vi "View_SUTR_FITS.vi"() -> ()   [LabVIEW 2012]
panel:
  in  "Autosave":bool
  in  "Default Res Directory":path=path "C:/DATA-RESULTS"
  out "error out 2":errorcluster
  in  "Normalize":bool
  in  "FF2":bool
  in  "FF1":bool
  in  "Read 1":bool
  in  "Read 2":bool
  out "Image 2":dbl[][](graph)
  in  "Files 2":i32(listbox)
  in  "Files 1":i32(listbox)
  out "int tome":sgl
  out "Median (ADU/sec)":dbl=6.0 format="%.3f"
  out "file name proc":string="Select file"
  out "Angle 1 ext (deg) 2":dbl=7.5
  out "Angle 1 ext (deg)":dbl=7.5
  out "dV (km/s)":dbl=-1.0193819817582153 format="%.3f"
  out "V (km/s) 2":dbl=7.5
  out "V (km/s) 1":dbl=7.5
  out "Temperature vs refractive index":cluster{dbl[], dbl[]}(graph)
  out "dOrder":dbl=-1.0193819817582153 format="%.3f"
  out "Order 2":dbl=1219.647194648069 format="%.3f"
  out "Order 1":dbl=1219.647194648069 format="%.3f"
  in  "Thickness":dbl=210.0 format="%.3f"
  in  "Wavelength":dbl=1.21 format="%.3f"
  in  "ORDERS/ANGLES":bool
  out "FOCUS 2":dbl[](array[numeric]) format="%.4f"
  out "Image 1":dbl[][](graph)
  in  "HDR PARAM":u16(ring) items=["FOCUS", "Etalons T"]
  out "AXIS 1":cluster{i32[], dbl[]}[](graph)
  out "Array 2":sgl[](array[numeric])
  out "Array":sgl[](array[numeric])
  out "AXIS 3":cluster{i32[], dbl[]}[](graph)
  out "FOCUS":dbl[][](array[numeric]) format="%.4f"
  out "Slice 4":dbl[][](graph)
  in  "Num refpix":u16=5
  in  "Remove refp?":bool
  out "STDEV selected":dbl[][](array[numeric]) format="%.4f"
  in  "Cols  sel":bool[](array[boolean])=[FALSE, TRUE, TRUE, FALSE]
  in  "Rows sel":bool[](array[boolean])=[TRUE, FALSE, FALSE, TRUE]
  out "Slice 3":dbl[][](graph)
  out "Slice 2":dbl[][](graph)
  in  "Init params colS":T1(array[cluster])=[{"initial amplitude"=33.77719364785919, "initial center"=49.70463978212081, "initial std devi"=0.19273176170627804, "offset"=90.64950374672406}, {"initial amplitude"=2584.714260893242, "initial center"=65.44858138705881, "initial std devi"=3.733463983192803, "offset"=284.499091020463}, {"initial amplitude"=780.252289907369, "initial center"=76.39143911404652, "initial std devi"=10.23938098152215, "offset"=81.40579465327467}, {"initial amplitude"=500.0, "initial center"=50.0, "initial std devi"=5.0, "offset"=0.0}]
  in  "Init params ROW":T1(array[cluster])=[{"initial amplitude"=1873.6125304433974, "initial center"=69.54989529124263, "initial std devi"=4.504262475173647, "offset"=252.28578992831524}, {"initial amplitude"=19.137742970969033, "initial center"=37.10397468007118, "initial std devi"=78.15537278387357, "offset"=38.82421297074018}, {"initial amplitude"=19.04875576622036, "initial center"=99.0, "initial std devi"=197.98265411656024, "offset"=62.014220893292794}, {"initial amplitude"=1000.0, "initial center"=50.0, "initial std devi"=5.0, "offset"=0.0}]
  in  "files":string[](array[string])
  in  "Read":bool
  out "Amplitude 2":dbl[][](array[numeric]) format="%.4f"
  out "STDEV 2":dbl[][](array[numeric]) format="%.4f"
  out "center 2":dbl[][](array[numeric]) format="%.4f"
  in  "initial guess COL":T2={"initial amplitude"=nan, "initial center"=nan, "initial std devi"=nan, "offset"=nan}
  out "center":dbl[][](array[numeric]) format="%.4f"
  out "STDEV":dbl[][](array[numeric]) format="%.4f"
  out "Amplitude":dbl[][](array[numeric]) format="%.4f"
  in  "error in (no error)":errorcluster
  in  "Process":bool
  in  "STOP":bool
  in  "Strip length":i32=600
  in  "Fit Gauss?":bool
  out "proc file #":i32
  in  "Select flatfield":u16(ring) items=["Std", "Read from disk", "Average  files"]
  in  "Norm?":bool
  out "Slice 7":dbl[][](graph)
  in  "FF array":dbl[][](array[numeric])=array1024x1024[1048576 elements] format="%.4f"
  out "Slice 6":dbl[][](graph)
  in  "Select file":string="Select file"
  out "Numeric":i32=3
  out "STDEV":dbl[][](graph)=[[3.80922583304428, 3.817188088612178, 3.977756374635943, 3.709975839173165, 4.204670281550964, 4.066080878455446, 4.561354633571724, 4.5262390212577985, 4.558772835455342, 4.581136884063742, 4.521486316852289, 4.971843226595924, 4.90608258535995, 5.27696401550079, 5.111911508066236, 5.170141203091181, 4.890928111688745, 4.907247135437398, 4.848191242418806, 4.83809156293769], [9.711095280614401, 9.971289019821658, 9.788245843410733, 9.923357541329326, 9.745666322543594, 9.786236649177065, 9.511348120785584, 9.373091410919924, 9.304927522805341, 9.10012745113379, 9.146622952912985, 8.993768484218087, 8.956214514109512, 8.674866890194615, 8.719154141237079, 8.611851720736974, 7.701630409119083, 7.651212652849094, 7.609036134707259, 7.603366762011219], [4.893862283261521, 3.912348921910702, 4.287711111176547, 3.968009269163568, 4.42781957244485, 4.444836685027503, 4.741397672118246, 4.721056037339747, 4.626346526841245, 4.919177778951065, 5.100781252748569, 5.5392420746888495, 5.539933224601394, 5.6020059507282385, 5.808813620501355, 6.182585147680958, 5.756524829207016, 5.473299468339225, 5.511785993835031, 5.18370376288494], [9.258933828121483, 9.191747417698833, 9.041217540948582, 9.413425961872695, 8.829487668253286, 9.160443411114333, 9.114654291796361, 8.72041762857734, 8.959900586090964, 8.636980944545334, 9.046089389007006, 8.887693711855636, 8.875586055417067, 8.921953916385833, 8.9718505032208, 9.04963948163129, 9.904011705941352, 9.675772758013501, 9.638785423011441, 9.552602582469593]]
  in  "parameter bounds":T3={"amp min"=0.0, "amp max"=20000.0, "center min"=0.0, "center max"=200.0, "deviation min"=-inf, "deviation max"=100.0, "offset min"=0.0, "offset max"=20000.0}
  out "STDV":dbl=9.552602582469593
  out "Position":dbl=49.896376621079575
  out "Amplitude":dbl=1955.4840499678983
  in  "Selection length":i32=200
  out "Slice 4":dbl[](graph)
  in  "initial guess ROW":T2={"initial amplitude"=nan, "initial center"=nan, "initial std devi"=nan, "offset"=nan}
  out "STDV":dbl[][](array[numeric])=[[3.80922583304428, 9.711095280614401, 4.893862283261521, 9.258933828121483], [3.817188088612178, 9.971289019821658, 3.912348921910702, 9.191747417698833], [3.977756374635943, 9.788245843410733, 4.287711111176547, 9.041217540948582], [3.709975839173165, 9.923357541329326, 3.968009269163568, 9.413425961872695], [4.204670281550964, 9.745666322543594, 4.42781957244485, 8.829487668253286], [4.066080878455446, 9.786236649177065, 4.444836685027503, 9.160443411114333], [4.561354633571724, 9.511348120785584, 4.741397672118246, 9.114654291796361], [4.5262390212577985, 9.373091410919924, 4.721056037339747, 8.72041762857734], [4.558772835455342, 9.304927522805341, 4.626346526841245, 8.959900586090964], [4.581136884063742, 9.10012745113379, 4.919177778951065, 8.636980944545334], [4.521486316852289, 9.146622952912985, 5.100781252748569, 9.046089389007006], [4.971843226595924, 8.993768484218087, 5.5392420746888495, 8.887693711855636], [4.90608258535995, 8.956214514109512, 5.539933224601394, 8.875586055417067], [5.27696401550079, 8.674866890194615, 5.6020059507282385, 8.921953916385833], [5.111911508066236, 8.719154141237079, 5.808813620501355, 8.9718505032208], [5.170141203091181, 8.611851720736974, 6.182585147680958, 9.04963948163129], [4.890928111688745, 7.701630409119083, 5.756524829207016, 9.904011705941352], [4.907247135437398, 7.651212652849094, 5.473299468339225, 9.675772758013501], [4.848191242418806, 7.609036134707259, 5.511785993835031, 9.638785423011441], [4.83809156293769, 7.603366762011219, 5.18370376288494, 9.552602582469593]]
  out "Peak position":dbl[][](array[numeric])=[[47.66372822279346, 45.737706176461124, 32.064423476273895, 41.26378980520465], [48.037887071447074, 44.121616415233404, 29.0359957584797, 42.88856881625823], [47.46412751971739, 43.40189101127855, 28.315113746919998, 42.853423144990614], [47.23633903151997, 43.98331127448147, 28.17624968549179, 43.20820023705084], [47.11670684274625, 43.43988511102371, 27.74805501482961, 43.138657897597355], [46.93922903400806, 43.9466885921773, 27.747501552953953, 43.29781271217172], [46.983170601290446, 43.4674057822943, 27.349010989971706, 43.4928736930594], [46.87826650279293, 43.73656484581372, 27.231418867922137, 43.59027544271928], [46.794602213066604, 43.80697609235037, 27.219441141475325, 43.86228314076525], [46.547609840673196, 43.49560932641496, 26.737210482499357, 43.83683218582205], [46.50275300580495, 43.93616768488781, 26.586165471065954, 44.24335733899606], [46.3894955614418, 43.74599122414512, 26.43758155462442, 44.18898136177602], [46.216839101721845, 44.127049565224574, 25.990860317183685, 44.52332837815359], [46.17676540353349, 43.92341806193053, 25.796393903324972, 44.59364842655686], [45.94651003970945, 44.243386449383074, 25.67343920426777, 44.94522728573687], [46.038982620545305, 43.96184867410636, 25.099486713825282, 45.28759471092761], [42.07400933436385, 46.63026758012912, 20.913656675675835, 49.256809286246366], [41.8831791471293, 46.71508407353966, 20.458660051313952, 49.58491224283602], [41.70930139549427, 46.95675849721172, 20.21435561030008, 49.95477829486535], [41.571263488082245, 46.859185888986325, 20.01183300897636, 49.896376621079575]]
  out "Amplitude":dbl[][](array[numeric])=[[2105.8622124215794, 1639.2467702622673, 2142.5270817793817, 1911.2610434851829], [2120.0504394951727, 1630.518269247327, 2157.8793469310863, 1968.0887445364817], [2074.081974979694, 1636.7175569641458, 2051.291440379497, 2013.3151234716927], [2141.4467291327323, 1637.469594377443, 2097.2888406416005, 1963.261978839169], [2066.222742080296, 1675.75453156014, 1978.306748333681, 2039.902099411284], [2067.624264099335, 1649.5982827860123, 1974.9594809186055, 2007.8700226013175], [1930.3219711177662, 1671.664946884232, 1963.7304764864682, 1990.0291865018387], [1934.7065510066398, 1695.403255048172, 1857.3519938646368, 2087.6349072163557], [2010.3064992166367, 1739.9324821026587, 1938.6975619656757, 2061.5356631230625], [1973.3790444228753, 1724.343555695147, 1890.962522743408, 2092.6867904284627], [1919.5387889965712, 1717.728353100013, 1795.3689110727476, 2025.044521524015], [1903.7560193442341, 1721.9496201330182, 1766.6216531350074, 2048.568854184652], [1930.4201947084764, 1755.9174293651708, 1799.1996079210312, 2065.114852823516], [1839.8756755419372, 1800.8508402487678, 1770.4507853937826, 2097.8006996715453], [1809.800026316876, 1800.6809656752282, 1725.998803512788, 2064.175733682101], [1803.9896118206118, 1802.8721092945568, 1680.5647072776162, 2085.0002611575646], [1908.2524607314188, 1994.827370627359, 1648.1186318102089, 1950.312562150539], [1902.2584452330298, 1968.3910778062084, 1640.241397396131, 1941.6845145841237], [1893.25547881938, 1983.5729978506592, 1613.927881985334, 1942.0488428956264], [1910.0015420712516, 1975.1048979055772, 1628.0987604984884, 1955.4840499678983]]
  out "Number of files":i32=20
  in  "Flatfield?":bool
  out "Sub Array":i32[][](array[numeric])
  out "Header":string="SIMPLE  =                    T / Files does conform to FITS standard            BITPIX  =                  -32 / Number of bits per data pixel                  NAXIS   =                    2 / Number of data axes                            NAXIS1  =                 1024 / Length of data axis 1                          NAXIS2  =                 1024 / Length of data axis 2                          EXTEND  =                      / FITS dataset may contain extensions            FOWLERNU=                    1 / Number of Fowler pairs                         OBJECT  =                      / Object Name                                    TELESCOP=                      / Telescope Name                                 INSTRUME=               'ZODI' / Instrument Name                                OBSERVER=                      / Observer Name                                  EQUINOX =                      / Coordinate Epoch                               NAME    ='111030412.5622.fits' / Filename                                       DATE    =         '03/04/2011' / Date                                           TIME    =           '12:56:22' / Time                                           JULIAN  =        2455625.24748 / Julian Date                                    INTTIME =             1.000000 / Integration Time                               FILTER  =                      / Filter                                         BSCALE  =                  1.0 / B Scale                                        BZERO   =                  0.0 / B Zero                                         CTYPE1  =             'PIXELS' / Axis type for dim 1 (e.g. RA)                  CTYPE2  =             'PIXELS' / Axis type for dim 2 (e.g. DEC)                 CRVAL1  =              0.00000 / Sky coord of 1st axis RA  (deg)                CRVAL2  =              0.00000 / Sky coord of 2nd axis DEC (deg)                CRPIX1  =                      / RA  ref point pixel location                   CRPIX2  =                      / DEC ref point pixel location                   TEMPA   =                 0.00 / Channel A                                      TEMPB   =                 0.00 / Channel B                                      TEMPC1  =                 0.00 / Etalon 1-250                                   TEMPC2  =                 0.00 / Etalon 2-210                                   TEMPC3  =                 0.00 / Filter Box                                     TEMPC4  =                 0.00 / Cold Plate                                     TEMPD1  =                 0.00 / Detector                                       TEMPD2  =                 0.00 / none                                           TEMPD3  =                 0.00 / none                                           TEMPD4  =                 0.00 / none                                           BIAS1   =                4.010 / BIAS 1                                         BIAS2   =                3.922 / BIAS 2                                         BIAS3   =                4.012 / BIAS 3                                         BIAS4   =                3.991 / BIAS 4                                         BIAS5   =                4.000 / BIAS 5                                         BIAS6   =                4.000 / BIAS 6                                         BIAS7   =                4.000 / BIAS 7                                         BIAS8   =                4.000 / BIAS 8                                         FOCUS1  =               -1.391 / Focus X Position                               FOCUS2  =                0.173 / Focus Y Position                               FOCUS3  =                0.020 / Focus Z Position                               FLTINDX =                    0 / Filter Index                                   FLTSTEP =                    0 / Filter Steps                                   FNAME   =                      / Filter Name                                    PRESSURE=          0.000000E+0 / Pressure                                       HEAT1   =                0.000 / Heater Etalon 1                                HEAT2   =                0.000 / Heater Etalon 2                                HEATD   =                0.000 / Heater Detector                                COMMENT =                                                                       END                                                                             "
  in  "Strip width":i32=20
  out "Slice 1":dbl[][](graph)
  out "Slice 2":dbl[](graph)=[-306.0, 4.0, -8.0, 11.0, -8.0, 226.0, 150.0, 188.0, 141.0, 154.0, 207.0, 167.0, 233.0, 226.0, 240.0, 292.0, 266.0, 288.0, 310.0, 280.0, 282.0, 336.0, 316.0, 206.0, 352.0, 136.0, 228.0, 300.0, 225.0, 284.0, 171.0, 136.0, 119.0, 150.0, 117.0, 114.0, 146.0, 142.0, 132.0, 102.0, 104.0, 113.0, 98.0, 110.0, 116.0, 70.0, 60.0, 66.0, 150.0, 132.0, 88.0, 96.0, 96.0, 138.0, 96.0, 185.0, 99.0, 98.0, 133.0, 110.0, 77.0, 74.0, 58.0, 72.0, 151.0, 106.0, 73.0, 116.0, 148.0, 150.0, 84.0, 98.0, 131.0, 122.0, 49.0, 128.0, 80.0, 80.0, 129.0, 165.0, 117.0, 107.0, 153.0, 118.0, 100.0, 97.0, 132.0, 181.0, 107.0, 105.0, 132.0, 138.0, 100.0, 69.0, 126.0, 118.0, 56.0, 94.0, 91.0, 119.0, 70.0, 86.0, 68.0, 108.0, 117.0, 176.0, 72.0, 102.0, 120.0, 138.0, 114.0, 130.0, 98.0, 121.0, 134.0, 103.0, 127.0, 109.0, 119.0, 210.0, 148.0, 134.0, 169.0, 122.0, 116.0, 126.0, 152.0, 92.0, 96.0, 218.0, 168.0, 228.0, 199.0, 197.0, 81.0, 168.0, 186.0, 169.0, 219.0, 184.0, 231.0, 200.0, 298.0, 296.0, 384.0, 262.0, 288.0, 514.0, 462.0, 442.0, 444.0, 342.0, 446.0, 592.0, 631.0, 696.0, 537.0, 796.0, 1097.0, 1056.0, 1286.0, 1415.0, 2354.0, 1398.0, 1502.0, 1508.0, 2106.0, 1889.0, 2272.0, 1350.0, 1890.0, 2253.0, 2489.0, 2663.0, 1860.0, 1565.0, 1630.0, 1408.0, 1197.0, 1240.0, 1414.0, 1125.0, 998.0, 932.0, 1024.0, 727.0, 776.0, 843.0, 627.0, 540.0, 442.0, 447.0, 413.0, 403.0, 308.0, 246.0, 302.0, 325.0, 389.0, 327.0, 244.0, 342.0, 235.0, 270.0, 350.0, 312.0, 232.0, 332.0, 240.0, 306.0, 210.0, 186.0, 236.0, 179.0, 216.0, 180.0, 240.0, 132.0, 249.0, 185.0, 194.0, 219.0, 109.0, 268.0, 301.0, 117.0, 167.0, 183.0, 64.0, 106.0, 174.0, 146.0, 161.0, 99.0, 114.0, 147.0, 93.0, 171.0, 120.0, 100.0, 165.0, 144.0, 216.0, 145.0, 75.0, 85.0, 108.0, 110.0, 158.0, 75.0, 128.0, 102.0, 150.0, 138.0, 101.0, 135.0, 104.0, 240.0, 157.0, 112.0, 115.0, 80.0, 76.0, 81.0, 127.0, 114.0, 82.0, 98.0, 110.0, 140.0, 116.0, 119.0, 145.0, 89.0, 176.0, 107.0, 214.0, 141.0, 61.0, 120.0, 118.0, 140.0, 112.0, 103.0, 30.0, 125.0, 151.0, 150.0, 162.0, 126.0, 92.0, 115.0, 73.0, 158.0, 150.0, 111.0, 124.0, 146.0, 81.0, 284.0, 154.0, 169.0, 155.0, 138.0, 124.0, 153.0, 96.0, 178.0, 170.0, 130.0, 139.0, 122.0, 103.0, -37.0, 122.0, 155.0, 106.0, 65.0, 79.0, 102.0, 117.0, 92.0, 64.0, 95.0, 96.0, 11.0, 116.0, 95.0, 119.0, 108.0, 63.0, 197.0, 118.0, 62.0, 50.0, 82.0, 77.0, 178.0, 110.0, 71.0, 62.0, 100.0, 75.0, 125.0, 70.0, 100.0, 148.0, 125.0, 97.0, 119.0, 140.0, 82.0, 144.0, 126.0, 74.0, 64.0, 62.0, 116.0, 90.0, 93.0, 110.0, 60.0, 84.0, 141.0, 43.0, 42.0, 90.0, 140.0, 98.0, 58.0, 119.0, 103.0, 136.0, 138.0, 70.0, 103.0, 115.0, 82.0, 97.0, 98.0, 100.0, 68.0, 105.0, 99.0, 84.0, 77.0, 88.0, 94.0, 192.0, 79.0, 131.0, 112.0, 88.0, 131.0, 62.0, 96.0, 148.0, 81.0, 108.0, 53.0, 75.0, 124.0, 111.0, 116.0, 137.0, 67.0, 113.0, 96.0, 60.0, 46.0, 119.0, 98.0, 130.0, 137.0, 178.0, 82.0, 43.0, 116.0, 143.0, 116.0, 107.0, 146.0, 121.0, 100.0, 101.0, 150.0, 155.0, 106.0, 75.0, 65.0, 92.0, 84.0, 68.0, 102.0, 98.0, 64.0, 123.0, 82.0, 109.0, 106.0, 101.0, 68.0, 95.0, 88.0, 97.0, 92.0, 79.0, 98.0, 57.0, 117.0, 89.0, 146.0, 41.0, 110.0, 85.0, 110.0, 134.0, 152.0, 60.0, 90.0, 183.0, 102.0, 110.0, 98.0, 144.0, 178.0, 144.0, 67.0, 119.0, 72.0, -25.0, 128.0, 78.0, 127.0, 105.0, 84.0, 91.0, 12.0, 93.0, 128.0, 157.0, 81.0, 48.0, 119.0, 115.0, 98.0, 123.0, 109.0, 94.0, 83.0, 74.0, 96.0, 148.0, 104.0, 123.0, 82.0, 46.0, 87.0, 74.0, 91.0, 54.0, 116.0, 147.0, 72.0, 157.0, 66.0, 110.0, 118.0, 60.0, 82.0, 126.0, 124.0, 124.0, 75.0, 138.0, 102.0, 92.0, 122.0, 58.0, 76.0, 63.0, 95.0, 74.0, 114.0, 88.0, 114.0, 56.0, 106.0, 89.0, 104.0, 68.0, 60.0, 121.0, 129.0, 118.0, 74.0, 188.0, 203.0, 162.0, 180.0, 81.0, 131.0, 77.0, 38.0, 66.0, 113.0, 139.0, 101.0, 113.0, 83.0, 70.0, 89.0, 103.0, 87.0, 86.0, 95.0, 78.0, 104.0, 148.0, 98.0, 62.0, 108.0, 52.0, 121.0, 112.0, 126.0, 68.0, 110.0, 77.0, 186.0, 117.0, 111.0, 103.0, 109.0, 157.0, 120.0, 116.0, 49.0, 12.0, 84.0, 144.0, 64.0, 72.0, 90.0, 86.0, 122.0, 41.0, 102.0, 96.0, 145.0, 112.0, 56.0, 58.0, 103.0, 114.0, 85.0, 58.0, 72.0, 67.0, 155.0, 62.0, 80.0, 137.0, 70.0, 98.0, 76.0, 98.0, 113.0, 125.0, 112.0, 107.0, 140.0, 84.0, 95.0, 80.0, 95.0, 96.0, 131.0, 88.0, 108.0, 48.0, 64.0, 115.0, 69.0, 76.0, 154.0, 138.0, 79.0, 129.0, 122.0, 139.0, 89.0, 86.0, 143.0, 123.0, 104.0, 53.0, 82.0, 152.0, 102.0, 57.0, 119.0, 120.0, 74.0, 132.0, 63.0, 86.0, 125.0, 95.0, 110.0, 136.0, 81.0, 91.0, 97.0, 82.0, 63.0, 154.0, 123.0, 110.0, 79.0, 54.0, 104.0, 180.0, 102.0, 50.0, 144.0, 111.0, 42.0, 84.0, 99.0, 126.0, 73.0, 101.0, 116.0, 85.0, 107.0, 89.0, 37.0, 98.0, 112.0, 79.0, 106.0, 103.0, 179.0, 102.0, 78.0, 125.0, 104.0, 97.0, 84.0, 88.0, 136.0, 32.0, 79.0, 102.0, 84.0, 34.0, 108.0, 76.0, 38.0, 134.0, 69.0, 81.0, 103.0, 85.0, 129.0, 143.0, 71.0, 98.0, 94.0, 44.0, 81.0, 175.0, 35.0, 118.0, 84.0, 179.0, 89.0, 37.0, 90.0, 87.0, 84.0, 88.0, 46.0, 36.0, 92.0, 76.0, 68.0, 54.0, -39.0, 60.0, 45.0, 68.0, 88.0, 128.0, 160.0, 121.0, 60.0, 124.0, 49.0, 122.0, 109.0, 174.0, 103.0, 95.0, 105.0, 134.0, 77.0, 77.0, 78.0, 141.0, 36.0, 74.0, 121.0, 88.0, 74.0, 95.0, 110.0, 105.0, 174.0, 68.0, 136.0, 128.0, 66.0, 70.0, 40.0, 72.0, 92.0, 95.0, 97.0, 49.0, 153.0, 109.0, 70.0, 62.0, 60.0, 158.0, 79.0, 92.0, 161.0, 66.0, 67.0, 78.0, 96.0, 109.0, 51.0, 173.0, 108.0, 147.0, 183.0, 74.0, 94.0, 120.0, 80.0, 134.0, 89.0, 56.0, -16.0, 94.0, 90.0, 26.0, 124.0, 88.0, 88.0, 82.0, 56.0, 67.0, 93.0, 104.0, 82.0, 121.0, 84.0, 115.0, 46.0, 101.0, 77.0, 20.0, 108.0, 66.0, 88.0, 74.0, 66.0, 126.0, 130.0, 33.0, 104.0, 88.0, 129.0, 93.0, 91.0, 78.0, 31.0, 129.0, 73.0, 40.0, 105.0, 78.0, 80.0, 99.0, 114.0, 52.0, 108.0, 54.0, 63.0, 88.0, 99.0, 96.0, 116.0, 92.0, 84.0, 146.0, 71.0, 65.0, 106.0, 107.0, 133.0, 136.0, 109.0, 113.0, 73.0, 41.0, 90.0, 175.0, 81.0, 107.0, 134.0, 135.0, 104.0, 85.0, 121.0, 80.0, 109.0, 166.0, 147.0, 133.0, 117.0, 132.0, 154.0, 125.0, 124.0, 150.0, 200.0, 161.0, 126.0, 171.0, 266.0, 175.0, 177.0, 301.0, 265.0, 149.0, 143.0, 185.0, 299.0, 158.0, 120.0, 119.0, 255.0, 290.0, 245.0, 254.0, 309.0, 205.0, 224.0, 379.0, 343.0, 303.0, 316.0, 480.0, 435.0, 437.0, 410.0, 625.0, 508.0, 572.0, 872.0, 768.0, 1180.0, 1554.0, 1463.0, 1204.0, 1306.0, 1805.0, 1380.0, 1684.0, 1665.0, 2388.0, 1898.0, 1150.0, 1765.0, 1211.0, 1278.0, 1008.0, 755.0, 628.0, 505.0, 380.0, 509.0, 498.0, 455.0, 590.0, 512.0, 447.0, 285.0, 518.0, 373.0, 347.0, 317.0, 322.0, 335.0, 182.0, 205.0, 264.0, 179.0, 156.0, 290.0, 216.0, 180.0, 107.0, 66.0, 97.0, 100.0, 130.0, 148.0, 131.0, 97.0, 112.0, 125.0, 104.0, 157.0, 124.0, 154.0, 66.0, 113.0, 70.0, 83.0, 127.0, 97.0, 133.0, 80.0, 106.0, 69.0, 123.0, 128.0, 87.0, 116.0, 106.0, 124.0, 96.0, 61.0, 112.0, 69.0, 77.0, 43.0, 88.0, 138.0, 109.0, 102.0, 48.0, 56.0, 88.0, 44.0, 80.0, 106.0, 84.0, 59.0, 88.0, 72.0, 115.0, 82.0, 22.0, 57.0, 78.0, 100.0, 84.0, 79.0, 125.0, 91.0, 85.0, 106.0, -2.0, 0.0, -10.0, 1.0, 2.0, 0.0, 12.0, -14.0, 0.0, 186.0, 188.0, 100.0, 148.0, 52.0, 86.0, 80.0, 90.0, 64.0, 98.0, 80.0, 106.0, 102.0, 100.0, 136.0, 90.0, 40.0, 134.0, 74.0, 64.0, 120.0, 74.0, 134.0, 96.0, 62.0, 80.0, 102.0, 106.0, 58.0, 122.0, 100.0, 70.0, 126.0, 74.0, 80.0, 112.0, 44.0, 94.0, 118.0, 80.0, 114.0, 144.0, 86.0, 72.0, 102.0, 128.0, 88.0, 120.0, 94.0, 136.0, 146.0, 122.0, 134.0, 106.0, 160.0, 174.0, 204.0, 276.0, 280.0, 200.0, 334.0, 240.0, 220.0, 342.0, 302.0, 330.0, 250.0, 354.0, 268.0, 258.0, 236.0, 158.0, 194.0, 144.0, 218.0, 134.0, 130.0, 116.0, 80.0, 110.0, 126.0, 130.0, 120.0, 98.0, 130.0, 100.0, 148.0, 106.0, 98.0, 110.0, 128.0, 98.0, 72.0, 104.0, 108.0, 132.0, 104.0, 108.0, 66.0, 204.0, 104.0, 104.0, 114.0, 86.0, 104.0, 38.0, 128.0, 104.0, 100.0, 122.0, 72.0, 72.0, 122.0, 156.0, 140.0, 132.0, 148.0, 86.0, 72.0, 106.0, 122.0, 140.0, 68.0, 82.0, 110.0, 80.0, 130.0, 88.0, 98.0, 112.0, 136.0, 138.0, 224.0, 86.0, 82.0, 104.0, 36.0, 86.0, 82.0, 100.0, 108.0, 108.0, 140.0, 100.0, 162.0, 118.0, 92.0, 100.0, 134.0, 68.0, 114.0, 102.0, 154.0, 84.0, 96.0, 178.0, 116.0, 224.0, 132.0, 78.0, 166.0, 130.0, 142.0, 114.0, 144.0, 84.0, 76.0, 148.0, 278.0, 122.0, 208.0, 172.0, 174.0, 132.0, 82.0, 94.0, 124.0, 202.0, 134.0, 170.0, 176.0, 156.0, 160.0, 130.0, 260.0, 244.0, 164.0, 208.0, 330.0, 324.0, 286.0, 462.0, 460.0, 358.0, 298.0, 422.0, 496.0, 368.0, 356.0, 492.0, 636.0, 582.0, 912.0, 590.0, 728.0, 960.0, 1122.0, 1322.0, 1146.0, 1358.0, 1412.0, 1668.0, 1750.0, 1348.0, 1494.0, 1784.0, 1630.0, 2430.0, 2424.0, 2260.0, 2330.0, 2126.0, 1934.0, 2190.0, 1808.0, 2816.0, 1314.0, 1562.0, 944.0, 1196.0, 1498.0, 1230.0, 1150.0, 930.0, 856.0, 894.0, 738.0, 720.0, 714.0, 570.0, 602.0, 560.0, 482.0, 432.0, 392.0, 480.0, 290.0, 352.0, 378.0, 292.0, 252.0, 352.0, 286.0, 236.0, 280.0, 258.0, 186.0, 266.0, 310.0, 282.0, 212.0, 342.0, 232.0, 222.0, 208.0, 230.0, 174.0, 280.0, 196.0, 138.0, 232.0, 256.0, 132.0, 154.0, 166.0, 262.0, 220.0, 184.0, 130.0, 204.0, 150.0, 124.0, 158.0, 210.0, 190.0, 94.0, 154.0, 146.0, 126.0, 148.0, 110.0, 152.0, 198.0, 152.0, 168.0, 118.0, 80.0, 76.0, 124.0, 150.0, 130.0, 102.0, 122.0, 128.0, 162.0, 136.0, 96.0, 232.0, 154.0, 102.0, 150.0, 102.0, 96.0, 114.0, 118.0, 106.0, 166.0, 118.0, 144.0, 154.0, 200.0, 140.0, 54.0, 112.0, 106.0, 142.0, 108.0, 170.0, 138.0, 122.0, 120.0, 96.0, 92.0, 156.0, 120.0, 196.0, 130.0, 144.0, 138.0, 164.0, 64.0, 200.0, 166.0, 212.0, 162.0, 206.0, 148.0, 134.0, 128.0, 152.0, 180.0, 164.0, 194.0, 180.0, 168.0, 102.0, 146.0, 180.0, 152.0, 228.0, 132.0, 158.0, 126.0, 130.0, 170.0, 130.0, 128.0, 168.0, 92.0, 164.0, 164.0, 96.0, 130.0, 118.0, 104.0, 112.0, 162.0, 184.0, 140.0, 232.0, 68.0, 72.0, 146.0, 108.0, 96.0, 102.0, 114.0, 108.0, 152.0, 132.0, 124.0, 82.0, 126.0, 116.0, 96.0, 128.0, 48.0, 86.0, 96.0, 62.0, 156.0, 126.0, 118.0, 132.0, 150.0, 128.0, 64.0, 54.0, 44.0, 52.0, 76.0, 112.0, 156.0, 120.0, 138.0, 136.0, 128.0, 114.0, 86.0, 80.0, 94.0, 150.0, 110.0, 164.0, 64.0, 110.0, 74.0, 130.0, 114.0, 96.0, 114.0, 166.0, 144.0, 64.0, 98.0, 70.0, 92.0, 102.0, 130.0, 90.0, 82.0, 80.0, 68.0, 166.0, 84.0, 32.0, 100.0, 82.0, 110.0, 144.0, 72.0, 78.0, 208.0, 102.0, 144.0, 96.0, 106.0, 56.0, 96.0, 110.0, 82.0, 68.0, 112.0, 168.0, 124.0, 124.0, 42.0, 78.0, 114.0, 82.0, 134.0, 142.0, 122.0, 124.0, 84.0, 116.0, 96.0, 86.0, 106.0, 70.0, 92.0, 124.0, 142.0, 144.0, 80.0, 84.0, 70.0, 106.0, 152.0, 92.0, 50.0, 110.0, 90.0, 100.0, 98.0, 110.0, 82.0, 78.0, 94.0, 80.0, 88.0, 90.0, 90.0, 46.0, 86.0, 122.0, 60.0, 65.0, 120.0, 78.0, 80.0, 77.0, 88.0, 124.0, 98.0, 163.0, 94.0, 140.0, 84.0, 86.0, 152.0, 73.0, 111.0, 73.0, 77.0, 103.0, 96.0, 91.0, 163.0, 90.0, 96.0, 172.0, 94.0, 130.0, 88.0, 119.0, 47.0, 82.0, 135.0, 116.0, 84.0, 148.0, 68.0, 121.0, 57.0, 162.0, 95.0, 105.0, 51.0, 67.0, 108.0, 102.0, 210.0, 68.0, 109.0, 136.0, 50.0, 188.0, 188.0, 146.0, 132.0, 106.0, 111.0, 56.0, 113.0, 101.0, 108.0, 79.0, 134.0, 89.0, 102.0, 111.0, 92.0, 140.0, 120.0, 56.0, 112.0, 147.0, -31.0, 104.0, 125.0, 15.0, 104.0, 84.0, 77.0, 104.0, 52.0, 121.0, 145.0, 78.0, 125.0, 158.0, 120.0, 78.0, 129.0, 115.0, 102.0, 104.0, 96.0, 151.0, 107.0, 80.0, 108.0, 114.0, 144.0, 69.0, 100.0, 114.0, 137.0, 76.0, 137.0, 66.0, 148.0, 56.0, 156.0, 142.0, 121.0, 130.0, 135.0, 164.0, 120.0, 93.0, 153.0, 116.0, 121.0, 136.0, 90.0, 93.0, 115.0, 44.0, 141.0, 95.0, 96.0, 132.0, 144.0, 209.0, 99.0, 70.0, 128.0, 143.0, 62.0, 141.0, 140.0, 70.0, 107.0, 50.0, 63.0, 151.0, 118.0, 151.0, 71.0, 101.0, 83.0, 109.0, 111.0, 158.0, 86.0, 133.0, 175.0, 154.0, 129.0, 93.0, 76.0, 142.0, 88.0, 38.0, -30.0, 61.0, 117.0, 125.0, 106.0, 86.0, 140.0, 112.0, 165.0, 131.0, 156.0, 132.0, 115.0, 156.0, 146.0, 169.0, 92.0, 111.0, 115.0, 120.0, 116.0, 94.0, 64.0, 80.0, 118.0, 141.0, 43.0, 83.0, 92.0, 132.0, 127.0, 141.0, 119.0, 101.0, 89.0, 92.0, 141.0, 105.0, 141.0, 93.0, 105.0, 95.0, 155.0, 127.0, 85.0, 221.0, 149.0, 131.0, 140.0, 87.0, 56.0, 98.0, 121.0, 23.0, 102.0, 93.0, 101.0, 57.0, 79.0, 116.0, 29.0, 124.0, 63.0, 116.0, 172.0, 101.0, 108.0, 129.0, 121.0, 126.0, 74.0, 78.0, 162.0, 60.0, 78.0, 96.0, 117.0, 103.0, 146.0, 179.0, 256.0, 172.0, 179.0, 39.0, 59.0, 106.0, 77.0, 112.0, 136.0, 133.0, 105.0, 168.0, 166.0, 133.0, 147.0, 172.0, 135.0, 95.0, 76.0, 148.0, 63.0, 145.0, 182.0, 90.0, 107.0, 118.0, 150.0, 84.0, 78.0, 119.0, 158.0, 85.0, 53.0, 160.0, 134.0, 120.0, 134.0, 126.0, 229.0, 125.0, 128.0, 101.0, 132.0, 175.0, 127.0, 202.0, 151.0, 130.0, 108.0, 189.0, 157.0, 112.0, 231.0, 149.0, 193.0, 107.0, 143.0, 151.0, 138.0, 147.0, 123.0, 118.0, 276.0, 96.0, 127.0, 130.0, 151.0, 125.0, 114.0, 119.0, 106.0, 151.0, 129.0, 184.0, 125.0, 89.0, 166.0, 142.0, 133.0, 113.0, 96.0, 143.0, 167.0, 143.0, 216.0, 158.0, 80.0, 216.0, 44.0, 79.0, 123.0, 96.0, 140.0, 153.0, 118.0, 127.0, 119.0, 76.0, 146.0, 97.0, 115.0, 120.0, 129.0, 144.0, 80.0, 105.0, 98.0, 124.0, 111.0, 97.0, 138.0, 124.0, 128.0, 86.0, 113.0, 127.0, 123.0, 128.0, 108.0, 147.0, 108.0, 93.0, 113.0, 59.0, 134.0, 155.0, 108.0, 164.0, 109.0, 127.0, 182.0, 110.0, 180.0, 118.0, 66.0, 88.0, 161.0, 97.0, 175.0, 197.0, 197.0, 157.0, 133.0, 100.0, 130.0, 112.0, 110.0, 200.0, 185.0, 183.0, 144.0, 164.0, 140.0, 114.0, 147.0, 181.0, 267.0, 197.0, 172.0, 157.0, 236.0, 161.0, 209.0, 220.0, 262.0, 210.0, 318.0, 283.0, 173.0, 312.0, 252.0, 237.0, 112.0, 367.0, 343.0, 226.0, 352.0, 311.0, 292.0, 488.0, 539.0, 467.0, 476.0, 430.0, 523.0, 361.0, 558.0, 542.0, 569.0, 788.0, 668.0, 948.0, 709.0, 1137.0, 906.0, 1089.0, 1344.0, 1373.0, 1444.0, 1630.0, 1584.0, 2442.0, 1776.0, 1876.0, 1835.0, 1217.0, 1901.0, 1929.0, 1557.0, 1665.0, 1196.0, 1374.0, 1362.0, 1216.0, 1006.0, 1012.0, 1299.0, 1141.0, 654.0, 905.0, 969.0, 719.0, 570.0, 635.0, 485.0, 693.0, 490.0, 414.0, 377.0, 321.0, 370.0, 372.0, 263.0, 284.0, 197.0, 143.0, 267.0, 263.0, 247.0, 202.0, 293.0, 241.0, 242.0, 147.0, 142.0, 184.0, 191.0, 164.0, 151.0, 160.0, 115.0, 127.0, 178.0, 180.0, 105.0, 221.0, 139.0, 71.0, 130.0, 146.0, 111.0, 93.0, 148.0, 56.0, 56.0, 104.0, 75.0, 113.0, 65.0, 5.0, -8.0, 9.0, -1.0]
  in  "Color Table":u16(ring)=3 items=["blue color", "infrared color", "weird c-table", "Unchanged"]
  in  "pattern (all files)":string="*.fits"
  in  "path":path=path "C:/DATA/20110304/series_focus_IN_150um"
  out "Input File:":path=path "C:/DATA/20110304/series_focus_IN_150um/111030412.5622.fits"
  out "Image":dbl[][](graph)
  # "A1"
  # "RIGHT"
  # "TOP"
  # "A2"
  # "A3"
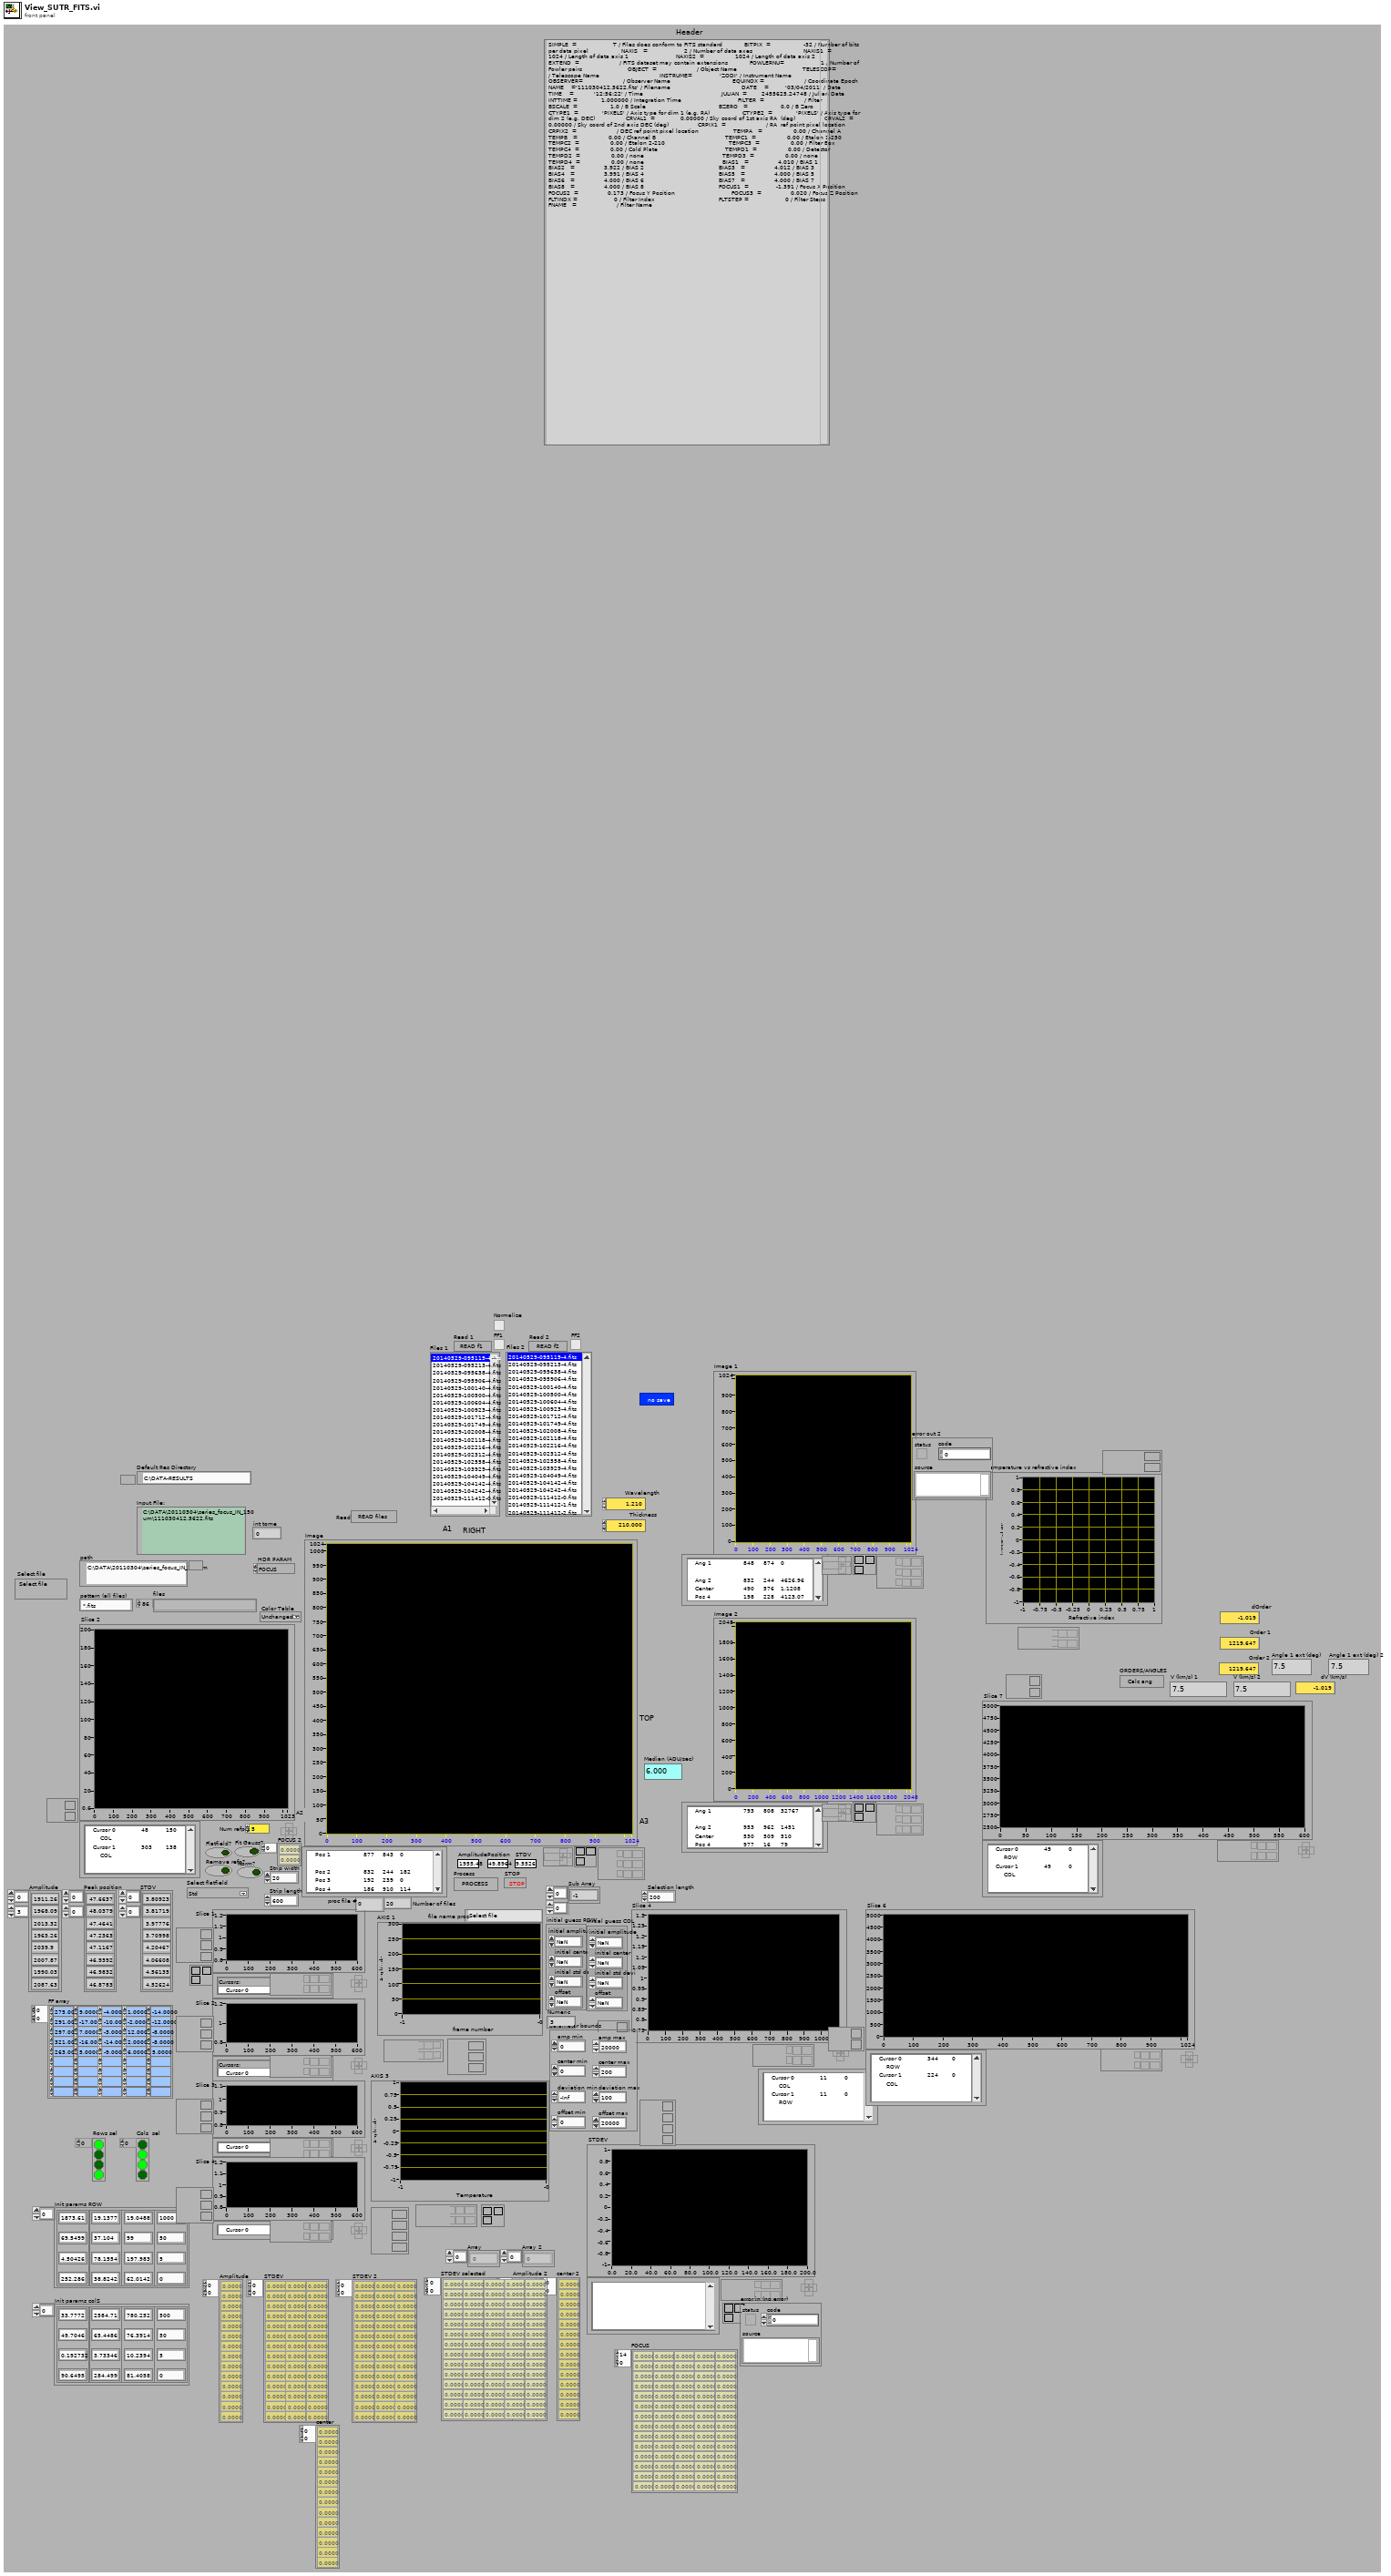
[diagram p1: front panel]
types:
  T1 = cluster{"initial amplitude":dbl, "initial center":dbl, "initial std devi":dbl, "offset":dbl}[]
  T2 = cluster{"initial amplitude":dbl, "initial center":dbl, "initial std devi":dbl, "offset":dbl}
  T3 = cluster{"amp min":dbl, "amp max":dbl, "center min":dbl, "center max":dbl, "deviation min":dbl, "deviation max":dbl, "offset min":dbl, "offset max":dbl}
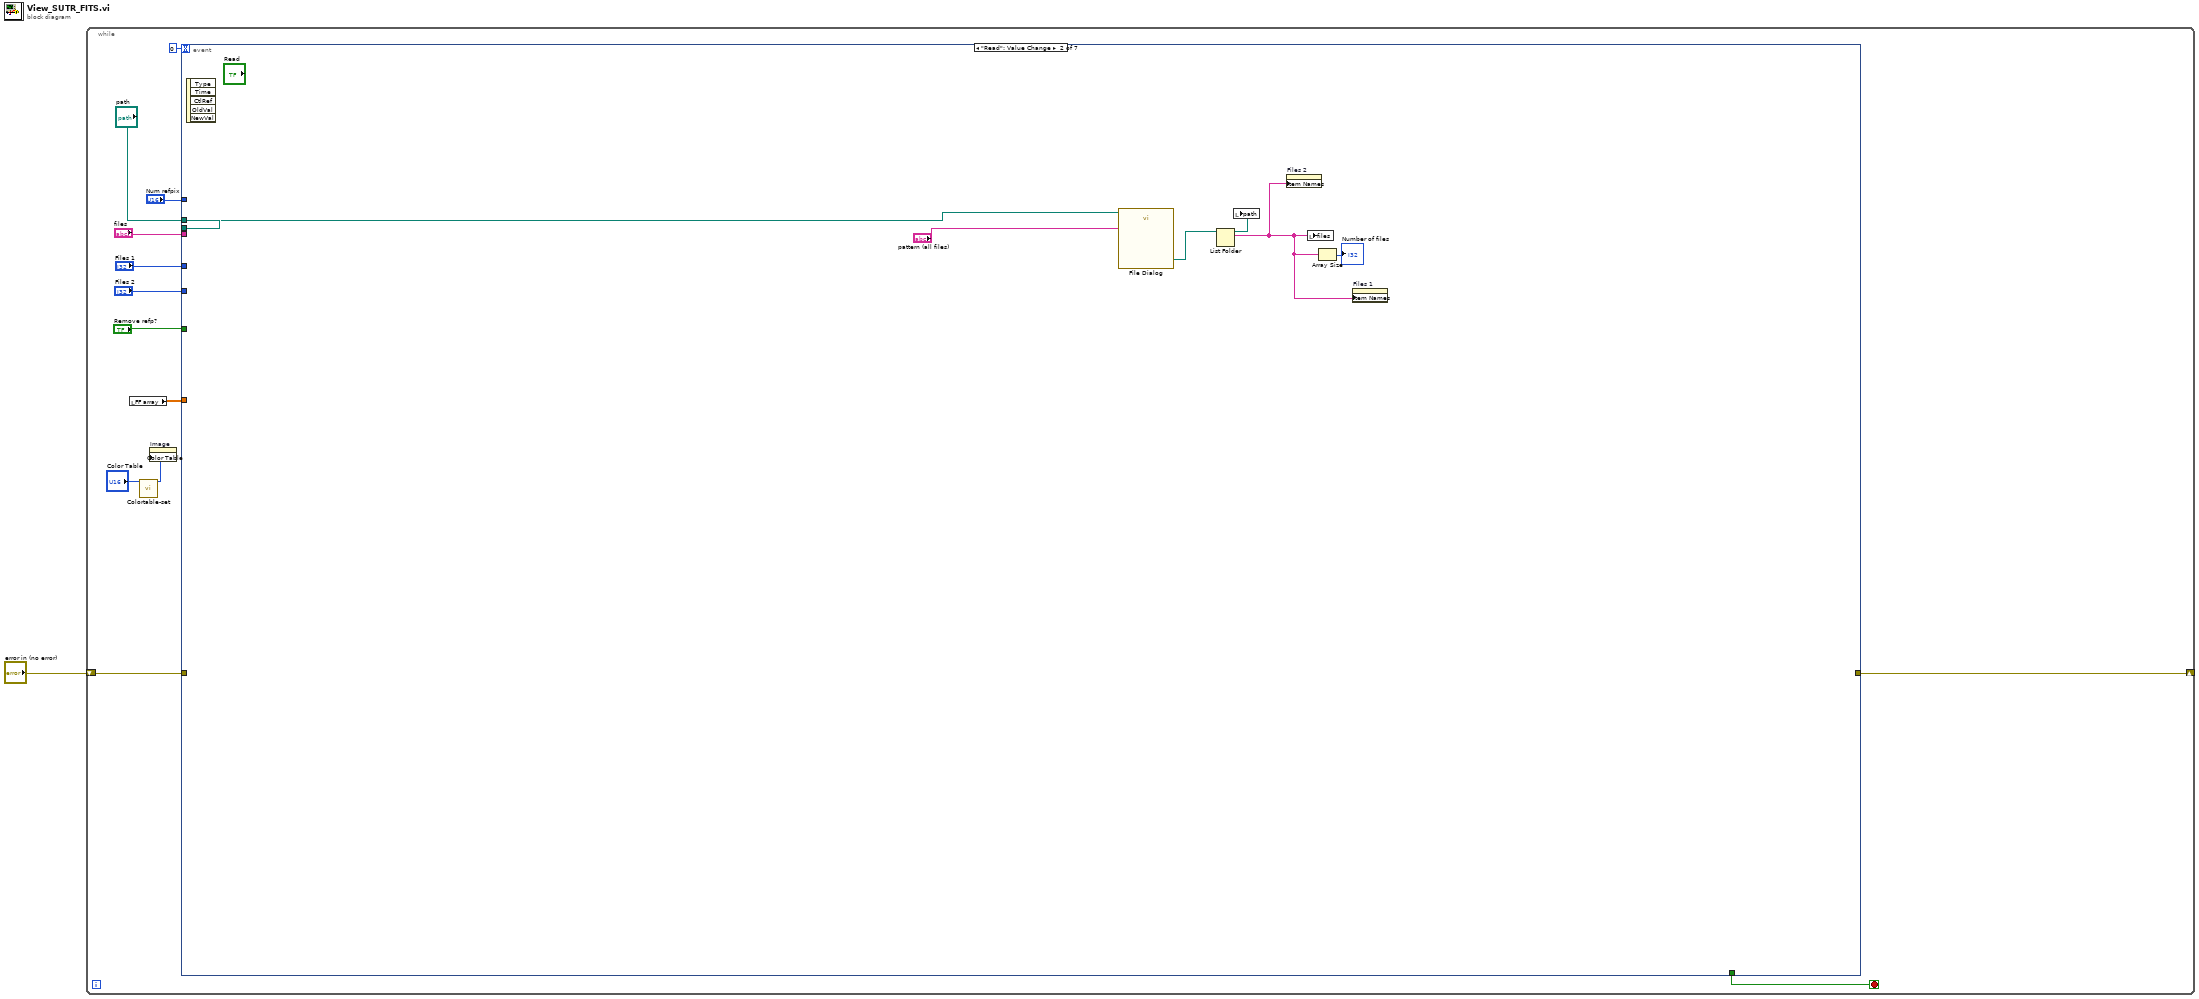
[diagram p0: block diagram]
diagram:
  n1 = while {
    shift-right: [w12] -> _
    shift-left: "error in (no error)" -> [w13]
    stop <- w14 stop-if-true
    n2 = local read "FF array"() -> (w3:dbl[][])
    n3 = call "Colortable-set.vi"("Color Table"="Color Table") -> ("Color table"=w8:u32[])  [unwired: 10 in]
    n4 = property on="Image" class="IntGraph (strict)"("Color Table"=w8) -> ()  [unwired: 2 in, 2 out]
    n5 = event shown="[1] \"Read\": Value Change" {
      selector: _ -> [_ _ _ _ _ _ _]
      dyn-events: _ -> [_ _ _ _ _ _ _]
      timeout: 0 -> [_ _ _ _ _ _ _]
      tunnel: "path" -> [_ _ w49 w234 _ _ _]
      tunnel: "files" -> [_ _ w48 w235 _ w318 w348]
      tunnel: ["STOP" _ _ _ _ _ _] -> w14